vi "CRYO_MASTER_FULL_RUN2.vi"() -> ()   [LabVIEW 2017] (continued)
                n236 = invoke class="TabCtl (strict)" method="Get Image"(error in=errorcluster {"status"=FALSE, "code"=0, "source"=""} ("error in (no error)")) -> (error out=w473:errorcluster, "image data"=w475:T23)  [unwired: 5 in, 4 out]
                n237 = Build Path(base path=w484, name or relative path=w477) -> (appended path=w476:path)
                n238 = call <vilib>:"Write PNG File.vi"("error in (no error)"=w473, "image data"=w475, "path to PNG file"=w476) -> ("error out"=w471:errorcluster)  [unwired: 7 in, 1 out]
              }
            }
            n239 = local write "error out (frontpanel screenshots)"(w464) -> ()
          }
          frame #5 {
            n240 = flat-sequence {
              tunnel: w488 -> [w491]
              tunnel: [w491] -> w487
              tunnel: w489 -> [w506]
              tunnel: w487 -> [w494]
              tunnel: [w493] -> w486
              tunnel: w485 -> [w492]
              frame #0 {
                n241 = property class="TabCtl (strict)"("Val(Sgnl)"=T1."DMMs" ("Value (Signaling)")) -> ()  [unwired: 2 in, 2 out]
              }
              frame #1 {
                w504 = "_" ("string")
                n242 = local read "Cycle #"() -> (w502:u32)
                n243 = call "LV_UNIXTIME.vi"("current time"=w494) -> ("date/time string"=w505:string)  [unwired: 9 in, 1 out]
                n244 = Format Value(format string="%06d", value (0)=w502) -> (output string=w501:string)  [unwired: 1 in]
                n245 = Concatenate Strings(w492, w505, w504, w501, w504, "page6.png" ("string")) -> (w499:string)
                n246 = invoke class="TabCtl (strict)" method="Get Image"(error in=errorcluster {"status"=FALSE, "code"=0, "source"=""} ("error in (no error)")) -> (error out=w495:errorcluster, "image data"=w497:T23)  [unwired: 5 in, 4 out]
                n247 = Build Path(base path=w506, name or relative path=w499) -> (appended path=w498:path)
                n248 = call <vilib>:"Write PNG File.vi"("error in (no error)"=w495, "image data"=w497, "path to PNG file"=w498) -> ("error out"=w493:errorcluster)  [unwired: 7 in, 1 out]
              }
            }
            n249 = local write "error out (frontpanel screenshots)"(w486) -> ()
          }
          frame #6 {
            n250 = flat-sequence {
              tunnel: w510 -> [w513]
              tunnel: [w513] -> w509
              tunnel: w511 -> [w528]
              tunnel: w509 -> [w516]
              tunnel: [w515] -> w508
              tunnel: w507 -> [w514]
              frame #0 {
                n251 = property class="TabCtl (strict)"("Val(Sgnl)"=T1."DIAGRAM" ("Value (Signaling)")) -> ()  [unwired: 2 in, 2 out]
              }
              frame #1 {
                w526 = "_" ("string")
                n252 = local read "Cycle #"() -> (w524:u32)
                n253 = Format Value(format string="%06d", value (0)=w524) -> (output string=w523:string)  [unwired: 1 in]
                n254 = call "LV_UNIXTIME.vi"("current time"=w516) -> ("date/time string"=w527:string)  [unwired: 9 in, 1 out]
                n255 = Concatenate Strings(w514, w527, w526, w523, w526, "page7.png" ("string")) -> (w521:string)
                n256 = invoke class="TabCtl (strict)" method="Get Image"(error in=errorcluster {"status"=FALSE, "code"=0, "source"=""} ("error in (no error)")) -> (error out=w517:errorcluster, "image data"=w519:T23)  [unwired: 5 in, 4 out]
                n257 = Build Path(base path=w528, name or relative path=w521) -> (appended path=w520:path)
                n258 = call <vilib>:"Write PNG File.vi"("error in (no error)"=w517, "image data"=w519, "path to PNG file"=w520) -> ("error out"=w515:errorcluster)  [unwired: 7 in, 1 out]
              }
            }
            n259 = local write "error out (frontpanel screenshots)"(w508) -> ()
          }
          frame #7 {
            n260 = flat-sequence {
              tunnel: w532 -> [w535]
              tunnel: [w535] -> w531
              tunnel: w533 -> [w550]
              tunnel: w531 -> [w538]
              tunnel: [w537] -> w530
              tunnel: w529 -> [w536]
              frame #0 {
                n261 = property class="TabCtl (strict)"("Val(Sgnl)"=T1."CHF" ("Value (Signaling)")) -> ()  [unwired: 2 in, 2 out]
              }
              frame #1 {
                w548 = "_" ("string")
                n262 = local read "Cycle #"() -> (w546:u32)
                n263 = Format Value(format string="%06d", value (0)=w546) -> (output string=w545:string)  [unwired: 1 in]
                n264 = call "LV_UNIXTIME.vi"("current time"=w538) -> ("date/time string"=w549:string)  [unwired: 9 in, 1 out]
                n265 = Concatenate Strings(w536, w549, w548, w545, w548, "page8.png" ("string")) -> (w543:string)
                n266 = invoke class="TabCtl (strict)" method="Get Image"(error in=errorcluster {"status"=FALSE, "code"=0, "source"=""} ("error in (no error)")) -> (error out=w539:errorcluster, "image data"=w541:T23)  [unwired: 5 in, 4 out]
                n267 = Build Path(base path=w550, name or relative path=w543) -> (appended path=w542:path)
                n268 = call <vilib>:"Write PNG File.vi"("error in (no error)"=w539, "image data"=w541, "path to PNG file"=w542) -> ("error out"=w537:errorcluster)  [unwired: 7 in, 1 out]
              }
            }
            n269 = local write "error out (frontpanel screenshots)"(w530) -> ()
          }
          frame #8 {
            n270 = flat-sequence {
              tunnel: w554 -> [w557]
              tunnel: [w557] -> w553
              tunnel: w555 -> [w572]
              tunnel: w553 -> [w560]
              tunnel: [w559] -> w552
              tunnel: w551 -> [w558]
              frame #0 {
                n271 = property class="TabCtl (strict)"("Val(Sgnl)"=T1."(Plc. hld.)" ("Value (Signaling)")) -> ()  [unwired: 2 in, 2 out]
              }
              frame #1 {
                w570 = "_" ("string")
                n272 = local read "Cycle #"() -> (w568:u32)
                n273 = Format Value(format string="%06d", value (0)=w568) -> (output string=w567:string)  [unwired: 1 in]
                n274 = call "LV_UNIXTIME.vi"("current time"=w560) -> ("date/time string"=w571:string)  [unwired: 9 in, 1 out]
                n275 = Concatenate Strings(w558, w571, w570, w567, w570, "page8.png" ("string")) -> (w565:string)
                n276 = invoke class="TabCtl (strict)" method="Get Image"(error in=errorcluster {"status"=FALSE, "code"=0, "source"=""} ("error in (no error)")) -> (error out=w561:errorcluster, "image data"=w563:T23)  [unwired: 5 in, 4 out]
                n277 = Build Path(base path=w572, name or relative path=w565) -> (appended path=w564:path)
                n278 = call <vilib>:"Write PNG File.vi"("error in (no error)"=w561, "image data"=w563, "path to PNG file"=w564) -> ("error out"=w559:errorcluster)  [unwired: 7 in, 1 out]
              }
            }
            n279 = local write "error out (frontpanel screenshots)"(w552) -> ()
          }
          frame #9 {
            n280 = local write "Frontpanel screenshots"(FALSE ("Frontpanel screenshots")) -> ()
          }
        }
        "error out (frontpanel screenshots)" <- w371
        n281 = property class="TabCtl (strict)"("Val(Sgnl)"=w369) -> ()  [unwired: 2 in, 2 out]
      }
      event "Stop Button": Value Change {
        n282 = event-data() -> ()  [unwired: 1 in, 3 out]
      }
    }
    n283 = Wait (ms)(milliseconds to wait=u32 123) -> ()  [unwired: 1 out]
  }
  n284 = while {
    stop <- w579 stop-if-true
    n285 = event shown="[6] \"Take Screenshot! 1\": Value Change" {
      selector: _ -> [_ _ _ _ _ _ _ _ _ _ _]
      dyn-events: _ -> [_ _ _ _ _ _ _ _ _ _ _]
      timeout: _ -> [_ _ _ _ _ _ _ _ _ _ _]
      tunnel: [_ _ _ _ _ _ _ _ _ _ TRUE] -> w579
      tunnel: [errorcluster {"status"=FALSE, "code"=0, "source"=""} ("error out") w583 _ _ _ _ w713 w730 w747 w764 errorcluster {"status"=FALSE, "code"=0, "source"=""} ("error out")] -> w575
      event Timeout {
        n286 = event-data() -> ()  [unwired: 1 in, 3 out]
      }
      event "log/linear 1": Value Change {
        n287 = event-data() -> ()  [unwired: 1 in, 6 out]
        n288 = flat-sequence {
          tunnel: [w584] -> w583
          frame #0 {
            n289 = Boolean To (0,1)(Boolean="log/linear 1") -> (0, 1=w589:i16)
            n290 = control-ref of="Graph 1"() -> (w585:refnum<vi>)
            n291 = property class="XYGraph (strict)"(reference=w585, error in=errorcluster {"status"=FALSE, "code"=0, "source"=""} ("error in (no error)"), "YScale.Mapping Mode"=w589) -> (error out=w587:errorcluster)  [unwired: 1 out]
            n292 = control-ref of="error out (USB6210)"() -> (w588:refnum<vi>)
            n293 = property class="Clust (strict)"(reference=w588, "Val(Sgnl)"=w587) -> (error out=w584:errorcluster)  [unwired: 1 in, 1 out]
          }
        }
      }
      event "log/linear 2": Value Change {
        n294 = event-data() -> ()  [unwired: 1 in, 6 out]
        n295 = flat-sequence {
          frame #0 {
            n296 = Boolean To (0,1)(Boolean="log/linear 2") -> (0, 1=w595:i16)
            n297 = control-ref of="Graph 2"() -> (w593:refnum<vi>)
            n298 = property class="XYGraph (strict)"(reference=w593, error in=errorcluster {"status"=FALSE, "code"=0, "source"=""} ("error in (no error)"), "YScale.Mapping Mode"=w595) -> (error out=w594:errorcluster)  [unwired: 1 out]
            n299 = control-ref of="error out (USB6210)"() -> (w592:refnum<vi>)
            n300 = property class="Clust (strict)"(reference=w592, "Value"=w594) -> ()  [unwired: 1 in, 2 out]
          }
        }
      }
      event "log/linear 3": Value Change {
        n301 = event-data() -> ()  [unwired: 1 in, 6 out]
        n302 = flat-sequence {
          frame #0 {
            n303 = Boolean To (0,1)(Boolean="log/linear 3") -> (0, 1=w601:i16)
            n304 = control-ref of="Graph 3"() -> (w597:refnum<vi>)
            n305 = property class="XYGraph (strict)"(reference=w597, error in=errorcluster {"status"=FALSE, "code"=0, "source"=""} ("error in (no error)"), "YScale.Mapping Mode"=w601) -> (error out=w600:errorcluster)  [unwired: 1 out]
            n306 = control-ref of="error out (USB6210)"() -> (w599:refnum<vi>)
            n307 = property class="Clust (strict)"(reference=w599, "Value"=w600) -> ()  [unwired: 1 in, 2 out]
          }
        }
      }
      event "log/linear 4": Value Change {
        n308 = event-data() -> ()  [unwired: 1 in, 6 out]
        n309 = flat-sequence {
          frame #0 {
            n310 = Boolean To (0,1)(Boolean="log/linear 4") -> (0, 1=w607:i16)
            n311 = control-ref of="Graph 4"() -> (w603:refnum<vi>)
            n312 = property class="XYGraph (strict)"(reference=w603, error in=errorcluster {"status"=FALSE, "code"=0, "source"=""} ("error in (no error)"), "YScale.Mapping Mode"=w607) -> (error out=w606:errorcluster)  [unwired: 1 out]
            n313 = control-ref of="error out (USB6210)"() -> (w605:refnum<vi>)
            n314 = property class="Clust (strict)"(reference=w605, "Value"=w606) -> ()  [unwired: 1 in, 2 out]
          }
        }
      }
      event "Plot selecter LSI218(1)\n    1      2     3     4", "Plot selecter LSI218(2)\n    1      2     3     4", "Plot selecter (USB6210)\n    1      2     3     4", "Plot selecter LSI336 \n     1      2     3     4", "Plot selecter (USB6218)\n    1      2     3     4": Value Change {
        n315 = event-data() -> ()  [unwired: 1 in, 6 out]
        n316 = local read "All Labels (USB6210)"() -> (w625:string[])
        n317 = local read "All Labels (USB6218)"() -> (w614:string[])
        n318 = local read "Labels LSI218 (1)"() -> (w627:string[])
        n319 = local read "Labels LSI218 (2)"() -> (w628:string[])
        n320 = local read "Labels LSI336"() -> (w620:string[])
        n321 = call "BuildPlotLegends_LSI218.vi"("Plot selecter (2)\n    1      2     3     5"="Plot selecter LSI218(2)\n    1      2     3     4", "Plot selecter (1)\n    1      2     3     4"="Plot selecter LSI218(1)\n    1      2     3     4", "Labels (2)"=w628, "Labels (1)"=w627) -> ("Series 4"=w638:string[], "Series 3"=w636:string[], "Series 2"=w634:string[], "Series 1"=w632:string[])  [unwired: 4 in]
        n322 = call "BuildPlotLegends.vi"("Plot selecter \n    1      2     3     4"="Plot selecter (USB6210)\n    1      2     3     4", "AllLabels"=w625) -> ("Series 4"=w637:string[], "Series 3"=w635:string[], "Series 2"=w633:string[], "Series 1"=w631:string[])  [unwired: 6 in]
        n323 = call "BuildPlotLegends.vi"("Plot selecter \n    1      2     3     4"="Plot selecter LSI336 \n     1      2     3     4", "AllLabels"=w620) -> ("Series 4"=w615:string[], "Series 3"=w616:string[], "Series 2"=w617:string[], "Series 1"=w618:string[])  [unwired: 6 in]
        n324 = call "BuildPlotLegends.vi"("Plot selecter \n    1      2     3     4"="Plot selecter (USB6218)\n    1      2     3     4", "AllLabels"=w614) -> ("Series 4"=w610:string[], "Series 3"=w609:string[], "Series 2"=w611:string[], "Series 1"=w612:string[])  [unwired: 6 in]
        n325 = Build Array (concatenate)(w633, w634, w617, w611) -> (w622:string[])
        "Series 2" <- w622
        n326 = Build Array (concatenate)(w635, w636, w616, w609) -> (w623:string[])
        "Series 3" <- w623
        n327 = Build Array (concatenate)(w637, w638, w615, w610) -> (w624:string[])
        "Series 4" <- w624
        n328 = Build Array (concatenate)(w631, w632, w618, w612) -> (w621:string[])
        "Series 1" <- w621
        n329 = stacked-sequence {
          tunnel: [w648 _ _ _] -> w642
          tunnel: [_ w666 _ _] -> w643
          tunnel: [_ _ w683 _] -> w641
          tunnel: [_ _ _ w700] -> w640
          tunnel: w621 -> [w646 _ _ _]
          tunnel: w622 -> [_ w664 _ _]
          tunnel: w623 -> [_ _ w681 _]
          tunnel: w624 -> [_ _ _ w698]
          frame #0 {
            n330 = Array Size(array=w646) -> (size(s)=w650:i32)
            n331 = control-ref of="Graph 1"() -> (w644:refnum<vi>)
            n332 = property class="XYGraph (strict)"(reference=w644) -> ("LegNumRows"=w645:u32)  [unwired: 1 in, 2 out]
            n333 = for {
              N: w645 -> [_]
              tunnel: w644 -> [w659]
              shift-right: [w657] -> w649
              shift-left: errorcluster {"status"=FALSE, "code"=0, "source"=""} ("error in (no error)") -> [w658]
              i -> [w661]
              n334 = property class="XYGraph (strict)"(reference=w659, error in=w658, "Active Plot"=w661, "Plot.Plot Name"="") -> (error out=w657:errorcluster)  [unwired: 1 out]
            }
            n335 = for {
              N: w650 -> [_]
              tunnel: w644 -> [w655]
              shift-right: [w653] -> w648
              shift-left: w649 -> [w654]
              tunnel: w646 -> [w652] mode=indexing
              i -> [w656]
              n336 = property class="XYGraph (strict)"(reference=w655, error in=w654, "Active Plot"=w656, "Plot.Plot Name"=w652, "Plot.Visible?"=TRUE ("Plot.Visible")) -> (error out=w653:errorcluster)  [unwired: 1 out]
            }
          }
          frame #1 {
            n337 = Array Size(array=w664) -> (size(s)=w668:i32)
            n338 = control-ref of="Graph 2"() -> (w663:refnum<vi>)
            n339 = property class="XYGraph (strict)"(reference=w663) -> ("LegNumRows"=w662:u32)  [unwired: 1 in, 2 out]
            n340 = for {
              N: w662 -> [_]
              shift-right: [w675] -> w667
              shift-left: errorcluster {"status"=FALSE, "code"=0, "source"=""} ("error in (no error)") -> [w676]
              tunnel: w663 -> [w674]
              i -> [w678]
              n341 = property class="XYGraph (strict)"(reference=w674, error in=w676, "Active Plot"=w678, "Plot.Plot Name"="") -> (error out=w675:errorcluster)  [unwired: 1 out]
            }
            n342 = for {
              N: w668 -> [_]
              shift-right: [w671] -> w666
              shift-left: w667 -> [w672]
              tunnel: w664 -> [w670] mode=indexing
              tunnel: w663 -> [w669]
              i -> [w673]
              n343 = property class="XYGraph (strict)"(reference=w669, error in=w672, "Active Plot"=w673, "Plot.Plot Name"=w670) -> (error out=w671:errorcluster)  [unwired: 1 out]
            }
          }
          frame #2 {
            n344 = Array Size(array=w681) -> (size(s)=w685:i32)
            n345 = control-ref of="Graph 3"() -> (w679:refnum<vi>)
            n346 = property class="XYGraph (strict)"(reference=w679) -> ("LegNumRows"=w680:u32)  [unwired: 1 in, 2 out]
            n347 = for {
              N: w680 -> [_]
              tunnel: w679 -> [w693]
              shift-right: [w691] -> w684
              shift-left: errorcluster {"status"=FALSE, "code"=0, "source"=""} ("error in (no error)") -> [w692]
              i -> [w695]
              n348 = property class="XYGraph (strict)"(reference=w693, error in=w692, "Active Plot"=w695, "Plot.Plot Name"="") -> (error out=w691:errorcluster)  [unwired: 1 out]
            }
            n349 = for {
              N: w685 -> [_]
              tunnel: w679 -> [w689]
              shift-right: [w687] -> w683
              shift-left: w684 -> [w688]
              tunnel: w681 -> [w686] mode=indexing
              i -> [w690]
              n350 = property class="XYGraph (strict)"(reference=w689, error in=w688, "Active Plot"=w690, "Plot.Plot Name"=w686) -> (error out=w687:errorcluster)  [unwired: 1 out]
            }
          }
          frame #3 {
            n351 = Array Size(array=w698) -> (size(s)=w702:i32)
            n352 = control-ref of="Graph 4"() -> (w696:refnum<vi>)
            n353 = property class="XYGraph (strict)"(reference=w696) -> ("LegNumRows"=w697:u32)  [unwired: 1 in, 2 out]
            n354 = for {
              N: w697 -> [_]
              tunnel: w696 -> [w710]
              shift-right: [w708] -> w701
              shift-left: errorcluster {"status"=FALSE, "code"=0, "source"=""} ("error in (no error)") -> [w709]
              i -> [w712]
              n355 = property class="XYGraph (strict)"(reference=w710, error in=w709, "Active Plot"=w712, "Plot.Plot Name"="") -> (error out=w708:errorcluster)  [unwired: 1 out]
            }
            n356 = for {
              N: w702 -> [_]
              tunnel: w696 -> [w706]
              shift-right: [w704] -> w700
              shift-left: w701 -> [w705]
              tunnel: w698 -> [w703] mode=indexing
              i -> [w707]
              n357 = property class="XYGraph (strict)"(reference=w706, error in=w705, "Active Plot"=w707, "Plot.Plot Name"=w703) -> (error out=w704:errorcluster)  [unwired: 1 out]
            }
          }
        }
        n358 = Merge Errors(w642, w643, w641, w640) -> (→"Plot errors":errorcluster)
      }
      event "Take Screenshot! 1": Value Change {
        n359 = event-data() -> ()  [unwired: 1 in, 6 out]
        n360 = flat-sequence {
          tunnel: [w714] -> w713
          frame #0 {
            n361 = flat-sequence {
              tunnel: [w715] -> w714
              frame #0 {
                w724 = "_" ("string")
                n362 = Get Date/Time In Seconds() -> (seconds since 1Jan1904=w721:timestamp)
                n363 = local read "RUN Identifier"() -> (w726:string)
                n364 = call "LV_UNIXTIME.vi"("current time"=w721) -> ("date/time string"=w725:string)  [unwired: 9 in, 1 out]
                n365 = control-ref of="Graph 1"() -> (w720:refnum<vi>)
                n366 = Concatenate Strings(w726, w724, w725, w724, "FIle suffix 1", ".png" ("string")) -> (w728:string)
                n367 = local read "Base Path"() -> (w727:path)
                n368 = invoke class="XYGraph (strict)" method="Get Image"(reference=w720, error in=errorcluster {"status"=FALSE, "code"=0, "source"=""} ("error in (no error)")) -> (error out=w716:errorcluster, "image data"=w719:T23)  [unwired: 4 in, 4 out]
                n369 = Build Path(base path=w727, name or relative path=w728) -> (appended path=w718:path)
                n370 = call <vilib>:"Write PNG File.vi"("error in (no error)"=w716, "image data"=w719, "path to PNG file"=w718) -> ("error out"=w715:errorcluster)  [unwired: 7 in, 1 out]
              }
              frame #1 {
                n371 = local write "Take Screenshot! 1"(FALSE ("Take Screenshot! 1")) -> ()
              }
            }
          }
        }
      }
      event "Take Screenshot! 2": Value Change {
        n372 = event-data() -> ()  [unwired: 1 in, 6 out]
        n373 = flat-sequence {
          tunnel: [w731] -> w730
          frame #0 {
            n374 = flat-sequence {
              tunnel: [w737] -> w731
              frame #0 {
                w741 = "_" ("string")
                n375 = Get Date/Time In Seconds() -> (seconds since 1Jan1904=w738:timestamp)
                n376 = local read "RUN Identifier"() -> (w743:string)
                n377 = call "LV_UNIXTIME.vi"("current time"=w738) -> ("date/time string"=w742:string)  [unwired: 9 in, 1 out]
                n378 = control-ref of="Graph 2"() -> (w732:refnum<vi>)
                n379 = Concatenate Strings(w743, w741, w742, w741, "FIle suffix 2", ".png" ("string")) -> (w745:string)
                n380 = local read "Base Path"() -> (w744:path)
                n381 = invoke class="XYGraph (strict)" method="Get Image"(reference=w732, error in=errorcluster {"status"=FALSE, "code"=0, "source"=""} ("error in (no error)")) -> (error out=w736:errorcluster, "image data"=w734:T23)  [unwired: 4 in, 4 out]
                n382 = Build Path(base path=w744, name or relative path=w745) -> (appended path=w733:path)
                n383 = call <vilib>:"Write PNG File.vi"("error in (no error)"=w736, "image data"=w734, "path to PNG file"=w733) -> ("error out"=w737:errorcluster)  [unwired: 7 in, 1 out]
              }
              frame #1 {
                n384 = local write "Take Screenshot! 2"(FALSE ("Take Screenshot! 1")) -> ()
              }
            }
          }
        }
      }
      event "Take Screenshot! 3": Value Change {
        n385 = event-data() -> ()  [unwired: 1 in, 6 out]
        n386 = flat-sequence {
          tunnel: [w748] -> w747
          frame #0 {
            n387 = flat-sequence {
              tunnel: [w750] -> w748
              frame #0 {
                w758 = "_" ("string")
                n388 = Get Date/Time In Seconds() -> (seconds since 1Jan1904=w756:timestamp)
                n389 = local read "RUN Identifier"() -> (w760:string)
                n390 = call "LV_UNIXTIME.vi"("current time"=w756) -> ("date/time string"=w759:string)  [unwired: 9 in, 1 out]
                n391 = control-ref of="Graph 3"() -> (w753:refnum<vi>)
                n392 = Concatenate Strings(w760, w758, w759, w758, "FIle suffix 3", ".png" ("string")) -> (w762:string)
                n393 = local read "Base Path"() -> (w761:path)
                n394 = invoke class="XYGraph (strict)" method="Get Image"(reference=w753, error in=errorcluster {"status"=FALSE, "code"=0, "source"=""} ("error in (no error)")) -> (error out=w751:errorcluster, "image data"=w749:T23)  [unwired: 4 in, 4 out]
                n395 = Build Path(base path=w761, name or relative path=w762) -> (appended path=w754:path)
                n396 = call <vilib>:"Write PNG File.vi"("error in (no error)"=w751, "image data"=w749, "path to PNG file"=w754) -> ("error out"=w750:errorcluster)  [unwired: 7 in, 1 out]
              }
              frame #1 {
                n397 = local write "Take Screenshot! 3"(FALSE ("Take Screenshot! 1")) -> ()
              }
            }
          }
        }
      }
      event "Take Screenshot! 4": Value Change {
        n398 = event-data() -> ()  [unwired: 1 in, 6 out]
        n399 = flat-sequence {
          tunnel: [w765] -> w764
          frame #0 {
            n400 = flat-sequence {
              tunnel: [w768] -> w765
              frame #0 {
                w775 = "_" ("string")
                n401 = Get Date/Time In Seconds() -> (seconds since 1Jan1904=w773:timestamp)
                n402 = local read "RUN Identifier"() -> (w777:string)
                n403 = call "LV_UNIXTIME.vi"("current time"=w773) -> ("date/time string"=w776:string)  [unwired: 9 in, 1 out]
                n404 = control-ref of="Graph 4"() -> (w769:refnum<vi>)
                n405 = Concatenate Strings(w777, w775, w776, w775, "FIle suffix 4", ".png" ("string")) -> (w779:string)
                n406 = local read "Base Path"() -> (w778:path)
                n407 = invoke class="XYGraph (strict)" method="Get Image"(reference=w769, error in=errorcluster {"status"=FALSE, "code"=0, "source"=""} ("error in (no error)")) -> (error out=w766:errorcluster, "image data"=w770:T23)  [unwired: 4 in, 4 out]
                n408 = Build Path(base path=w778, name or relative path=w779) -> (appended path=w771:path)
                n409 = call <vilib>:"Write PNG File.vi"("error in (no error)"=w766, "image data"=w770, "path to PNG file"=w771) -> ("error out"=w768:errorcluster)  [unwired: 7 in, 1 out]
              }
              frame #1 {
                n410 = local write "Take Screenshot! 4"(FALSE ("Take Screenshot! 1")) -> ()
              }
            }
          }
        }
      }
      event "Stop Button": Value Change {
        n411 = event-data() -> ()  [unwired: 1 in, 6 out]
      }
    }
    "error out (graph operations)" <- w575
    n412 = local write "Take Screenshot! 1"(FALSE ("Take Screenshot! 1")) -> ()
    n413 = local write "Take Screenshot! 2"(FALSE ("Take Screenshot! 1")) -> ()
    n414 = Wait (ms)(milliseconds to wait=u32 1000) -> ()  [unwired: 1 out]
    n415 = local write "Take Screenshot! 3"(FALSE ("Take Screenshot! 1")) -> ()
    n416 = local write "Take Screenshot! 4"(FALSE ("Take Screenshot! 1")) -> ()
  }
  n417 = while {
    i -> [w787]
    stop <- w784 stop-if-true
    n418 = Equal?(x=w787, y=0) -> (x = y?=w785:bool)
    n419 = case shown="True" w785 {
      frame False {
      }
      frame True {
        n420 = property on="Agilent\nIntialized?" class="Bool (strict)"("Val(Sgnl)"=FALSE ("Value (Signaling)")) -> ()  [unwired: 2 in, 2 out]
      }
    }
    n421 = Wait (ms)(milliseconds to wait=u32 123) -> ()  [unwired: 1 out]
    n422 = event shown="[4] \"V_lim_up (V)\", \"V_lim_low (V)\": Value Change" {
      selector: _ -> [_ _ _ _ _]
      dyn-events: _ -> [_ _ _ _ _]
      timeout: _ -> [_ _ _ _ _]
      tunnel: [FALSE ("Value (Signaling)") TRUE ("Value (Signaling)") _ _ _] -> w784
      tunnel: "VISA (Agilent 34402)" -> [_ _ w793 w796 _]
      event Timeout {
        n423 = event-data() -> ()  [unwired: 1 in, 3 out]
      }
      event "Stop Button": Value Change {
        n424 = event-data() -> ()  [unwired: 1 in, 3 out]
      }
      event "Initialize (Agilent)": Value Change {
        n425 = event-data() -> ()  [unwired: 1 in, 3 out]
        n426 = property on="Agilent\nIntialized?" class="Bool (strict)"("Val(Sgnl)"=TRUE ("Value (Signaling)")) -> ()  [unwired: 2 in, 2 out]
        n427 = call "Initialize.vi"("error in (no error)"=errorcluster {"status"=FALSE, "code"=0, "source"=""}, "VISA resource name"=w793) -> ("error out"=→"error out (Agilent)":errorcluster)  [unwired: 8 in, 1 out]
      }
      event "OUTPUT \nKenwood", "Kenwood set V (V)": Value Change {
        n428 = local read "Agilent\nIntialized?"() -> (w795:bool)
        n429 = event-data() -> ()  [unwired: 1 in, 3 out]
        n430 = case shown="True" w795 {
          tunnel: w796 -> [_ w802]
          frame False {
          }
          frame True {
            w804 = u16 0 items=["DC", "Sine", "Square", "Triangle", "Ramp", "Pulse", "Noise", "Sinc", "Negative Ramp", "Exponential Rise", "Exponential Fall", "Cardiac"] ("Waveform Function (1: Sine)")
            n431 = xnode "Formula"("X1"="Kenwood set V (V)") -> ("Result"=w797:dbl)  [unwired: 1 in, 1 out]
            n432 = call "Configure Standard Waveform.vi"("DC Offset (0.00 V)"=w797, "Frequency (1000 Hz)"=1.0, "error in (no error)"=errorcluster {"status"=FALSE, "code"=0, "source"=""}, "Amplitude (1)"=1.0, "Waveform Function (1: Sine)"=w804, "VISA resource name"=w802) -> ("error out"=w806:errorcluster, "VISA resource name out"=w807:refnum<visa-resource-name>)  [unwired: 4 in]
            n433 = call "Enable Output.vi"("error in (no error)"=w806, "Enable Output  (T: Enable)"="OUTPUT \nKenwood", "VISA resource name"=w807) -> ("error out"=w800:errorcluster)  [unwired: 7 in, 1 out]
            n434 = local write "error out (Agilent)"(w800) -> ()
          }
        }
      }
      event "V_lim_up (V)", "V_lim_low (V)": Value Change {
        n435 = event-data() -> ()  [unwired: 1 in, 3 out]
        n436 = property on="Kenwood set V (V)" class="DigNum (strict)"("Minimum"="V_lim_low (V)", "Maximum"="V_lim_up (V)") -> ()  [unwired: 2 in, 2 out]
      }
    }
  }
  n437 = while {
    stop <- w819 stop-if-true
    n438 = Wait (ms)(milliseconds to wait=u32 101) -> ()  [unwired: 1 out]
    n439 = event shown="[2] Timeout" {
      selector: _ -> [_ _ _]
      dyn-events: _ -> [_ _ _]
      timeout: _ -> [_ _ _]
      tunnel: [FALSE TRUE FALSE] -> w819
      event "Initialize (DMMs)": Value Change {
        w822 = T4 [] ("Value (Signaling)")
        n440 = event-data() -> ()  [unwired: 1 in, 3 out]
        n441 = property on="Graph DMMs 1" class="XYGraph (strict)"("Val(Sgnl)"=w822) -> ()  [unwired: 2 in, 2 out]
        n442 = property on="Graph DMMs 2" class="XYGraph (strict)"("Val(Sgnl)"=w822) -> ()  [unwired: 2 in, 2 out]
      }
      event "Stop Button": Value Change {
        n443 = event-data() -> ()  [unwired: 1 in, 3 out]
      }
      event Timeout {
        n444 = event-data() -> ()  [unwired: 1 in, 3 out]
      }
    }
  }
  n445 = Obtain Notifier(name (unnamed)="stop notifier", notification data type=w15, create if not found? (T)=w15, error in (no error)=errorcluster {"status"=FALSE, "code"=0, "source"=""}) -> (notifier out=w3:refnum<notifier>, error out=w2:errorcluster)  [unwired: 1 out]
  n446 = while {
    shift-right: [w922] -> w38
    shift-left: refnum<class "USBData.lvclass"> refnum ("USBData.lvclass") -> [w925]
    shift-right: [w918] -> w37
    shift-left: w4 -> [w924]
    tunnel: "Base Path" -> [w862]
    shift-right: [w900] -> w32
    shift-left: errorcluster {"status"=FALSE, "code"=0, "source"=""} ("error in (no error)") -> [w916]
    shift-right: [w901] -> w33
    shift-left: refnum<class "LSI218Data.lvclass"> refnum ("LSI218Data.lvclass") -> [w915]
    shift-right: [w888] -> w29
    shift-left: refnum<class "LSI336Data.lvclass"> refnum ("LSI336Data.lvclass") -> [w897]
    shift-right: [w887] -> w28
    shift-left: w19 -> [w896]
    shift-right: [w876] -> _
    shift-left: w4 -> [w877]
    shift-right: [w866] -> w23
    shift-left: refnum<class "USBData.lvclass"> refnum ("USBData.lvclass") -> [w874]
    shift-right: [w865] -> w22
    shift-left: errorcluster {"status"=FALSE, "code"=0, "source"=""} ("error in (no error)") -> [w873]
    shift-right: [w861] -> _
    shift-left: w19 -> [w860]
    tunnel: w3 -> [w829]
    tunnel: w2 -> [w828]
    tunnel: [w826] -> w11
    tunnel: [w825] -> w10
    i -> [w837]
    stop <- "Stop Button" stop-if-true
    w883 = u32 24 ("Number of Rows")
    w893 = T25 [] ("appended array")
    w910 = T25 [] ("appended array")
    n447 = local read "LSI218Settings(A-F)"() -> (w852:T3)
    n448 = control-ref of="Plot selecter LSI218(2)\n    1      2     3     4"() -> (w881:refnum<vi>)
    n449 = control-ref of="Plot selecter LSI218(1)\n    1      2     3     4"() -> (w882:refnum<vi>)
    n450 = control-ref of="Plot selecter LSI336 \n     1      2     3     4"() -> (w880:refnum<vi>)
    n451 = property on="Property Node" class="Arr (strict)"(reference=w881, "Number of Rows"=w883) -> ()  [unwired: 1 in, 2 out]
    n452 = property on="Property Node" class="Arr (strict)"(reference=w882, "Number of Rows"=w883) -> ()  [unwired: 1 in, 2 out]
    n453 = local read "LSI336Settings(X,Y)"() -> (w850:T3)
    n454 = Array Size(array=w852) -> (size(s)=w851:i32)
    n455 = property on="Property Node" class="Arr (strict)"(reference=w880, "Number of Rows"=u32 8) -> ()  [unwired: 1 in, 2 out]
    n456 = Multiply(x="Measurement Interval (s)", y=u32 1000) -> (x*y=w919:dbl)
    n457 = Wait (ms)(milliseconds to wait=w919) -> ()  [unwired: 1 out]
    n458 = for {
      N: w851 -> [_]
      tunnel: w852 -> [w936] mode=indexing
      tunnel: [w935] -> w848 mode=concatenating
      n459 = Unbundle By Name(w936) -> ("SensorLocations"=w935:T18)
    }
    n460 = for {
      tunnel: w850 -> [w934] mode=indexing
      tunnel: [w933] -> w849 mode=concatenating
      n461 = Unbundle By Name(w934) -> ("SensorLocations"=w933:T18)
    }
    n462 = Quotient & Remainder(x=w837, y="Screenshots interval") -> (x-y*floor(x/y)=w835:i64)  [unwired: 1 out]
    n463 = Equal?(x=w837, y=0) -> (x = y?=w830:bool)
    n464 = case shown="True" w830 {
      tunnel: w925 -> [w1991 w2014]
      tunnel: w924 -> [w1985 w2012]
      tunnel: w837 -> [w1976 _]
      tunnel: [w1983 w2009] -> w918
      tunnel: [w1980 w2008] -> w875
      tunnel: [w1981 w2007] -> w922
      tunnel: [w1971 w2002] -> w923
      tunnel: w862 -> [_ w2001]
      tunnel: [w1970 w1998] -> w857
      frame False {
        n465 = call-dynamic "USBData_measure.vi"("USBData in"=w1991, "DAQ sample #"=i64 5, "DAQ timeout"=100.0 ("DAQ timeout (def: 100)"), "MeasurementIndex"=w1976, "error in (no error)"=w1985, "save every ... measurements"="Record interval") -> ("USBData out"=w1990:refnum<class "USBData.lvclass">, "TimeMeasuremeent"=w1987:timestamp, "Status"=→"USB6210 Status":T6, "LastDataAcquired"=w1972:dbl[], "error out"=w1986:errorcluster)  [unwired: 3 in, 2 out]
        "Time of Last Measurement (USB6210)" <- w1987
        "Last Vol\n(USB6210)" <- w1972
        n466 = call-dynamic "USBData_convert.vi"("Save every ... measurements"="Record interval", "MeasurementIndex"=w1976, "error in (no error)"=w1986, "LastDataAcquired"=w1972, "TimeMeasuremeent"=w1987, "USBData in"=w1990) -> ("error out"=w1984:errorcluster, "LeakDet_FULL"=w1979:dbl, "LastDataConverted"=w1973:dbl[], "USBData out"=w1982:refnum<class "USBData.lvclass">)  [unwired: 2 in]
        n467 = call "USBData_read.vi"("USBData in"=w1982, "error in (no error)"=w1984) -> ("Status"=w1974:T6, "USBData out"=w1981:refnum<class "USBData.lvclass">, "Data"=w1980:T26, "Basic"=w1971:T27, "error out"=w1983:errorcluster)  [unwired: 2 in, 2 out]
        n468 = local write "USB6210 Status"(w1974) -> ()
        n469 = Unbundle By Name(w1971) -> ("ReadLeakDet?"=w1978:bool)
        n470 = Unbundle By Name(w1971) -> ("Labels"=w1970:string[])
        n471 = case shown="False" w1978 {
          tunnel: w1973 -> [w1992 w1995]
          tunnel: w1979 -> [_ w1994]
          tunnel: [w1992 w1993] -> w1977
          frame False {
          }
          frame True {
            n472 = Build Array (concatenate)(w1995, w1994) -> (w1993:dbl[])
          }
        }
        "Last Data \n(USB6210)" <- w1977
      }
      frame True {
        n473 = local read "RUN Identifier"() -> (w1996:string)
        n474 = call-dynamic "USBData_initialize.vi"("USBData in"=w2014, "SeriesSetting"="USB6210 Config", "BasePath"=w2001, "RunIdentifier"=w1996, "FileName"="InstName (USB6210)", "error in (no error)"=w2012) -> ("Status"=w1997:T6, "USBData out"=w2010:refnum<class "USBData.lvclass">, "error out"=w2011:errorcluster)  [unwired: 5 in, 2 out]
        n475 = local write "USB6210 Status"(w1997) -> ()
        n476 = call "USBData_read.vi"("USBData in"=w2010, "error in (no error)"=w2011) -> ("Status"=w2000:T6, "USBData out"=w2007:refnum<class "USBData.lvclass">, "Data"=w2008:T26, "Basic"=w2002:T27, "error out"=w2009:errorcluster)  [unwired: 2 in, 2 out]
        n477 = local write "USB6210 Status"(w2000) -> ()
        n478 = Unbundle By Name(w2002) -> ("ReadLeakDet?"=w2006:bool, "Labels"=w1998:string[])
        n479 = Array Size(array=w1998) -> (size(s)=w2005:i32)
        n480 = case shown="True" w2006 {
          tunnel: w2005 -> [w2015 w2017]
          tunnel: [w2015 w2016] -> w2003
          frame False {
          }
          frame True {
            n481 = Add(x=w2017, y=1) -> (x+y=w2016:i32)
          }
        }
        n482 = Initialize Array(TRUE ("Activate 2"), w2003) -> ()  [unwired: 1 out]
      }
    }
    "error out (USB6210)" <- w918
    n483 = case shown="False" w830 {
      tunnel: [w1507 w1534] -> w865
      tunnel: [w1504 w1533] -> w872
      tunnel: [w1505 w1532] -> w866
      tunnel: [w1496 w1527] -> w871
      tunnel: [w1495 w1525] -> _
      tunnel: w874 -> [w1494 w1523]
      tunnel: w862 -> [_ w1522]
      tunnel: w873 -> [w1493 w1521]
      tunnel: w837 -> [w1492 _]
      frame False {
        n484 = local read "Record interval"() -> (w1491:i64)
        n485 = call-dynamic "USBData_measure.vi"("USBData in"=w1494, "DAQ sample #"=i64 5, "DAQ timeout"=100.0 ("DAQ timeout (def: 100)"), "MeasurementIndex"=w1492, "error in (no error)"=w1493, "save every ... measurements"=w1491) -> ("USBData out"=w1513:refnum<class "USBData.lvclass">, "TimeMeasuremeent"=w1510:timestamp, "Status"=→"USB6218 Status":T6, "LastDataAcquired"=w1497:dbl[], "error out"=w1509:errorcluster)  [unwired: 3 in, 2 out]
        "Time of Last Measurement (USB6218)" <- w1510
        "Last Vol \n(USB6218)" <- w1497
        n486 = call-dynamic "USBData_convert.vi"("Save every ... measurements"=w1491, "MeasurementIndex"=w1492, "error in (no error)"=w1509, "LastDataAcquired"=w1497, "TimeMeasuremeent"=w1510, "USBData in"=w1513) -> ("error out"=w1508:errorcluster, "LeakDet_FULL"=w1503:dbl, "LastDataConverted"=w1498:dbl[], "USBData out"=w1506:refnum<class "USBData.lvclass">)  [unwired: 2 in]
        n487 = call "USBData_read.vi"("USBData in"=w1506, "error in (no error)"=w1508) -> ("Status"=w1499:T6, "USBData out"=w1505:refnum<class "USBData.lvclass">, "Data"=w1504:T26, "Basic"=w1496:T27, "error out"=w1507:errorcluster)  [unwired: 2 in, 2 out]
        n488 = local write "USB6218 Status"(w1499) -> ()
        n489 = Unbundle By Name(w1496) -> ("ReadLeakDet?"=w1502:bool)
        n490 = Unbundle By Name(w1496) -> ("Labels"=w1495:string[])
        n491 = case shown="True" w1502 {
          tunnel: w1498 -> [w1514 w1517]
          tunnel: w1503 -> [_ w1516]
          tunnel: [w1514 w1515] -> w1501
          frame False {
          }
          frame True {
            n492 = Build Array (concatenate)(w1517, w1516) -> (w1515:dbl[])
          }
        }
        "Last Data \n(USB6218)" <- w1501
      }
      frame True {
        n493 = local read "RUN Identifier"() -> (w1518:string)
        n494 = call-dynamic "USBData_initialize.vi"("USBData in"=w1523, "SeriesSetting"="USB6218 Config", "BasePath"=w1522, "RunIdentifier"=w1518, "FileName"="InstName (USB6218)", "error in (no error)"=w1521) -> ("Status"=w1519:T6, "USBData out"=w1535:refnum<class "USBData.lvclass">, "error out"=w1536:errorcluster)  [unwired: 5 in, 2 out]
        n495 = local write "USB6218 Status"(w1519) -> ()
        n496 = call "USBData_read.vi"("USBData in"=w1535, "error in (no error)"=w1536) -> ("Status"=w1526:T6, "USBData out"=w1532:refnum<class "USBData.lvclass">, "Data"=w1533:T26, "Basic"=w1527:T27, "error out"=w1534:errorcluster)  [unwired: 2 in, 2 out]
        n497 = local write "USB6218 Status"(w1526) -> ()
        n498 = Unbundle By Name(w1527) -> ("ReadLeakDet?"=w1531:bool, "Labels"=w1525:string[])
        n499 = Array Size(array=w1525) -> (size(s)=w1530:i32)
        n500 = case shown="True" w1531 {
          tunnel: w1530 -> [w1537 w1539]
          tunnel: [w1537 w1538] -> w1528
          frame False {
          }
          frame True {
            n501 = Add(x=w1539, y=1) -> (x+y=w1538:i32)
          }
        }
        n502 = Initialize Array(TRUE ("Activate 2"), w1528) -> ()  [unwired: 1 out]
      }
    }
    "error out (USB6218)" <- w865
    n503 = case shown="True" w830 {
      frame False {
      }
      frame True {
        n504 = local read "RUN label"() -> (w927:string)
        n505 = Get Date/Time In Seconds() -> (seconds since 1Jan1904=w931:timestamp)
        n506 = call "LV_UNIXTIME.vi"("current time"=w931) -> ("date/time string"=w930:string)  [unwired: 9 in, 1 out]
        n507 = Concatenate Strings(w930, "_" ("string"), w927) -> (→"RUN Identifier" →"RUN Identifier 2" →"RUN Identifier 3" →"RUN Identifier 4" →"RUN Identifier 5" →"RUN Identifier 6" →"RUN Identifier 7":string)
      }
    }
    n508 = Equal?(x=w835, y=i64 0) -> (x = y?=w832:bool)
    n509 = local read "LastData (LSI218)"() -> (w846:dbl[])
    n510 = local read "Last Data \nLSI336"() -> (w845:dbl[])
    n511 = And(x="Analog Out ON?", y=w830) -> (x .and. y?=w863:bool)
    n512 = case shown="True" w863 {
      tunnel: w862 -> [_ w1310]
      tunnel: [w1286 w1301] -> w861
      tunnel: w860 -> [w1286 w1300]
      frame False {
      }
      frame True {
        w1293 = "_raw" ("string")
        w1317 = 10.0 ("V_lim_max")
        w1316 = 0.0 ("V_lim_min")
        w1315 = -1 items=["Default"=-1, "RSE"=10083, "Differential"=10106, "Pseudodifferential"=12529] ("output terminal configuration")
        w1314 = 10348 items=["Volts"=10348, "From Custom Scale"=10065] ("units")
        n513 = local read "RUN Identifier"() -> (w1299:string)
        n514 = Concatenate Strings(w1299, "_AO" ("string")) -> (w1319:string)
        n515 = Concatenate Strings(w1299, "_", "USB_AOUT.csv" ("string")) -> (w1311:string)
        n516 = Array To Cluster(array="AOUT Labels") -> (cluster=w1297:T28)
        n517 = Unbundle By Name(w1297) -> ("AOUT Labels[0]"=w1296:string, "AOUT Labels[1]"=w1294:string)
        n518 = Build Path(base path=w1310, name or relative path=w1311) -> (appended path=w1307:path)
        n519 = Concatenate Strings(w1296, w1293) -> (w1295:string)
        n520 = Concatenate Strings(w1294, w1293) -> (w1292:string)
        n521 = Open/Create/Replace File(file path (use dialog)=w1307, operation (0:open)=T24."open or create") -> (refnum out=w1305:refnum<file>)  [unwired: 4 in, 2 out]
        n522 = Build Array(w1296, w1294, w1295, w1292) -> (w1303:string[])
        n523 = call "FileIntialize.vi"("Error In"=w1300, "Labels"=w1303, "refnum in"=w1305) -> ("Error Out"=w1302:errorcluster, "File Refnum"=→"File Refn USB AO":refnum<file>)  [unwired: 7 in]
        n524 = call <vilib>:"DAQmx Create Task.vi"("new task name"=w1319, "auto cleanup"=FALSE, "error in"=w1302) -> ("task out"=w1318:refnum<k21>, "error out"=w1320:errorcluster)  [unwired: 11 in]
        n525 = Index Array(array="AOUT assignment", index #1=0 ("index"), index #2=1 ("index")) -> (element #1=w1289:tag, element #2=w1287:tag)
        n526 = call-poly <vilib>:"DAQmx Create Virtual Channel.vi"("task in"=w1318, "maximum value"=w1317, "minimum value"=w1316, "output terminal configuration"=w1315, "physical channels"=w1289, "units"=w1314, "error in"=w1320) -> ("task out"=w1322:refnum<k21>, "error out"=w1323:errorcluster)  [unwired: 7 in]
        n527 = call-poly <vilib>:"DAQmx Create Virtual Channel.vi"("task in"=w1322, "maximum value"=w1317, "minimum value"=w1316, "physical channels"=w1287, "error in"=w1323) -> ("task out"=w1325:refnum<k21>, "error out"=w1324:errorcluster)  [unwired: 9 in]
        n528 = call <vilib>:"DAQmx Start Task.vi"("task/channels in"=w1325, "error in"=w1324) -> ("task out"=→"AO task out":refnum<k21>, "error out"=w1301:errorcluster)  [unwired: 12 in]
      }
    }
    "error out (USB6210/6218 AOUT)" <- w861
    n529 = And(x=w832, y="Automatic \nScreenshots?") -> (x .and. y?=w831:bool)
    n530 = Build Array (concatenate)(w846, w845) -> (w844:dbl[])
    "AllTemperatures" <- w844
    n531 = Build Array (concatenate)(w848, w849) -> (w847:T18)
    "TempSensorsLocations" <- w847
    n532 = case shown="True" w831 {
      frame False {
      }
      frame True {
        n533 = flat-sequence {
          frame #0 {
            n534 = property on="Frontpanel screenshots" class="Bool (strict)"("Val(Sgnl)"=TRUE ("Value (Signaling)")) -> ()  [unwired: 2 in, 2 out]
          }
        }
      }
    }
    n535 = flat-sequence {
      tunnel: w844 -> [w937]
      tunnel: w847 -> [w938]
      tunnel: w839 -> [w1190]
      tunnel: w838 -> [w1189]
      frame #0 {
        n536 = stacked-sequence {
          tunnel: w938 -> [w943 w948 w953 w958 w963 w968 w973 w978 w983 w988 w993 w998 w1003 w1008 w1013 w1018 w1023 w1028 w1033 w1038 w1043 w1048 w1053 w1058 w1063 w1068 w1073 w1078 w1083 w1088 w1093 w1098 w1103 w1108 w1113 w1118 w1123 w1128 w1133 w1138 w1143 w1148 w1153 w1158 w1163 w1168 w1173 w1178 w1183 w1188]
          tunnel: w937 -> [w941 w946 w951 w956 w961 w966 w971 w976 w981 w986 w991 w996 w1001 w1006 w1011 w1016 w1021 w1026 w1031 w1036 w1041 w1046 w1051 w1056 w1061 w1066 w1071 w1076 w1081 w1086 w1091 w1096 w1101 w1106 w1111 w1116 w1121 w1126 w1131 w1136 w1141 w1146 w1151 w1156 w1161 w1166 w1171 w1176 w1181 w1186]
          frame #0 {
            n537 = Search 1D Array(1D array=w943, element=T14."T3He1-1" ("SensorLocations")) -> (index of element=w940:i32)  [unwired: 1 in]
            n538 = Index Array(array=w941, index=w940) -> (element=→"T3He1-1":dbl)
          }
          frame #1 {
            n539 = Search 1D Array(1D array=w948, element=T14."T3He1-2" ("SensorLocations")) -> (index of element=w945:i32)  [unwired: 1 in]
            n540 = Index Array(array=w946, index=w945) -> (element=→"T3He1-2":dbl)
          }
          frame #2 {
            n541 = Search 1D Array(1D array=w953, element=T14."T3He1-3" ("SensorLocations")) -> (index of element=w950:i32)  [unwired: 1 in]
            n542 = Index Array(array=w951, index=w950) -> (element=→"T3He1-3":dbl)
          }
          frame #3 {
            n543 = Search 1D Array(1D array=w958, element=T14."T3He1-4" ("SensorLocations")) -> (index of element=w955:i32)  [unwired: 1 in]
            n544 = Index Array(array=w956, index=w955) -> (element=→"T3He1-4":dbl)
          }
          frame #4 {
            n545 = Search 1D Array(1D array=w963, element=T14."T3He2-1" ("SensorLocations")) -> (index of element=w960:i32)  [unwired: 1 in]
            n546 = Index Array(array=w961, index=w960) -> (element=→"T3He2-1":dbl)
          }
          frame #5 {
            n547 = Search 1D Array(1D array=w968, element=T14."T3He2-2" ("SensorLocations")) -> (index of element=w965:i32)  [unwired: 1 in]
            n548 = Index Array(array=w966, index=w965) -> (element=→"T3He2-2":dbl)
          }
          frame #6 {
            n549 = Search 1D Array(1D array=w973, element=T14."T3He3" ("SensorLocations")) -> (index of element=w970:i32)  [unwired: 1 in]
            n550 = Index Array(array=w971, index=w970) -> (element=→"T3He3":dbl)
          }
          frame #7 {
            n551 = Search 1D Array(1D array=w978, element=T14."T3He4" ("SensorLocations")) -> (index of element=w975:i32)  [unwired: 1 in]
            n552 = Index Array(array=w976, index=w975) -> (element=→"T3He4":dbl)
          }
          frame #8 {
            n553 = Search 1D Array(1D array=w983, element=T14."T3He5" ("SensorLocations")) -> (index of element=w980:i32)  [unwired: 1 in]
            n554 = Index Array(array=w981, index=w980) -> (element=→"T3He5":dbl)
          }
          frame #9 {
            n555 = Search 1D Array(1D array=w988, element=T14."T3He6-1" ("SensorLocations")) -> (index of element=w985:i32)  [unwired: 1 in]
            n556 = Index Array(array=w986, index=w985) -> (element=→"T3He6-1" →"T3He6-1/6-2 (HEX1)":dbl)
          }
          frame #10 {
            n557 = Search 1D Array(1D array=w993, element=T14."T3He6-2" ("SensorLocations")) -> (index of element=w990:i32)  [unwired: 1 in]
            n558 = Index Array(array=w991, index=w990) -> (element=→"T3He6-2" →"T3He6-1/6-2 (3He pot) 2":dbl)
          }
          frame #11 {
            n559 = Search 1D Array(1D array=w998, element=T14."T3He7-1" ("SensorLocations")) -> (index of element=w995:i32)  [unwired: 1 in]
            n560 = Index Array(array=w996, index=w995) -> (element=→"T3He7-1" →"T3He7-1/7-2 (HEX1)":dbl)
          }
          frame #12 {
            n561 = Search 1D Array(1D array=w1003, element=T14."T3He7-2" ("SensorLocations")) -> (index of element=w1000:i32)  [unwired: 1 in]
            n562 = Index Array(array=w1001, index=w1000) -> (element=→"T3He7-2" →"T3He7-1/6-2 (3He pot) 2":dbl)
          }
          frame #13 {
            n563 = Search 1D Array(1D array=w1008, element=T14."T3He8" ("SensorLocations")) -> (index of element=w1005:i32)  [unwired: 1 in]
            n564 = Index Array(array=w1006, index=w1005) -> (element=→"T3He8":dbl)
          }
          frame #14 {
            n565 = Search 1D Array(1D array=w1013, element=T14."T3He9" ("SensorLocations")) -> (index of element=w1010:i32)  [unwired: 1 in]
            n566 = Index Array(array=w1011, index=w1010) -> (element=→"T3He9":dbl)
          }
          frame #15 {
            n567 = Search 1D Array(1D array=w1018, element=T14."T3He10" ("SensorLocations")) -> (index of element=w1015:i32)  [unwired: 1 in]
            n568 = Index Array(array=w1016, index=w1015) -> (element=→"T3He10":dbl)
          }
          frame #16 {
            n569 = Search 1D Array(1D array=w1023, element=T14."T4He1" ("SensorLocations")) -> (index of element=w1020:i32)  [unwired: 1 in]
            n570 = Index Array(array=w1021, index=w1020) -> (element=→"T4He1" →"T4He1 (4K reservoir )":dbl)
          }
          frame #17 {
            n571 = Search 1D Array(1D array=w1028, element=T14."T4He2-1" ("SensorLocations")) -> (index of element=w1025:i32)  [unwired: 1 in]
            n572 = Index Array(array=w1026, index=w1025) -> (element=→"T4He2-1":dbl)
          }
          frame #18 {
            n573 = Search 1D Array(1D array=w1033, element=T14."T4He2-2" ("SensorLocations")) -> (index of element=w1030:i32)  [unwired: 1 in]
            n574 = Index Array(array=w1031, index=w1030) -> (element=→"T4He2-2":dbl)
          }
          frame #19 {
            n575 = Search 1D Array(1D array=w1038, element=T14."T4He3-1" ("SensorLocations")) -> (index of element=w1035:i32)  [unwired: 1 in]
            n576 = Index Array(array=w1036, index=w1035) -> (element=→"T4He3-1":dbl)
          }
          frame #20 {
            n577 = Search 1D Array(1D array=w1043, element=T14."T4He3-2" ("SensorLocations")) -> (index of element=w1040:i32)  [unwired: 1 in]
            n578 = Index Array(array=w1041, index=w1040) -> (element=→"T4He3-2":dbl)
          }
          frame #21 {
            n579 = Search 1D Array(1D array=w1048, element=T14."T4He3-3" ("SensorLocations")) -> (index of element=w1045:i32)  [unwired: 1 in]
            n580 = Index Array(array=w1046, index=w1045) -> (element=→"T4He3-3":dbl)
          }
          frame #22 {
            n581 = Search 1D Array(1D array=w1053, element=T14."T4He3-4" ("SensorLocations")) -> (index of element=w1050:i32)  [unwired: 1 in]
            n582 = Index Array(array=w1051, index=w1050) -> (element=→"T4He3-4":dbl)
          }
          frame #23 {
            n583 = Search 1D Array(1D array=w1058, element=T14."T4He4" ("SensorLocations")) -> (index of element=w1055:i32)  [unwired: 1 in]
            n584 = Index Array(array=w1056, index=w1055) -> (element=→"T4He4":dbl)
          }
          frame #24 {
            n585 = Search 1D Array(1D array=w1063, element=T14."T4He5" ("SensorLocations")) -> (index of element=w1060:i32)  [unwired: 1 in]
            n586 = Index Array(array=w1061, index=w1060) -> (element=→"T4He5":dbl)
          }
          frame #25 {
            n587 = Search 1D Array(1D array=w1068, element=T14."T4He6" ("SensorLocations")) -> (index of element=w1065:i32)  [unwired: 1 in]
            n588 = Index Array(array=w1066, index=w1065) -> (element=→"T4He6":dbl)
          }
          frame #26 {
            n589 = Search 1D Array(1D array=w1073, element=T14."T4He7" ("SensorLocations")) -> (index of element=w1070:i32)  [unwired: 1 in]
            n590 = Index Array(array=w1071, index=w1070) -> (element=→"T4He7":dbl)
          }
          frame #27 {
            n591 = Search 1D Array(1D array=w1078, element=T14."T4He8" ("SensorLocations")) -> (index of element=w1075:i32)  [unwired: 1 in]
            n592 = Index Array(array=w1076, index=w1075) -> (element=→"T4He8":dbl)
          }
          frame #28 {
            n593 = Search 1D Array(1D array=w1083, element=T14."T4He9" ("SensorLocations")) -> (index of element=w1080:i32)  [unwired: 1 in]
            n594 = Index Array(array=w1081, index=w1080) -> (element=→"T4He9":dbl)
          }
          frame #29 {
            n595 = Search 1D Array(1D array=w1088, element=T14."T4He10" ("SensorLocations")) -> (index of element=w1085:i32)  [unwired: 1 in]
            n596 = Index Array(array=w1086, index=w1085) -> (element=→"T4He10":dbl)
          }
          frame #30 {
            n597 = Search 1D Array(1D array=w1093, element=T14."T1K1" ("SensorLocations")) -> (index of element=w1090:i32)  [unwired: 1 in]
            n598 = Index Array(array=w1091, index=w1090) -> (element=→"T1K1":dbl)
          }
          frame #31 {
            n599 = Search 1D Array(1D array=w1098, element=T14."T1K2" ("SensorLocations")) -> (index of element=w1095:i32)  [unwired: 1 in]
            n600 = Index Array(array=w1096, index=w1095) -> (element=→"T1K2":dbl)
          }
          frame #32 {
            n601 = Search 1D Array(1D array=w1103, element=T14."T1K3-1" ("SensorLocations")) -> (index of element=w1100:i32)  [unwired: 1 in]
            n602 = Index Array(array=w1101, index=w1100) -> (element=→"T1K3-1" →"T1K3-1/3-2 (1K pot)":dbl)
          }
          frame #33 {
            n603 = Search 1D Array(1D array=w1108, element=T14."T1K3-2" ("SensorLocations")) -> (index of element=w1105:i32)  [unwired: 1 in]
            n604 = Index Array(array=w1106, index=w1105) -> (element=→"T1K3-2" →"T1K3-1/3-2 (1K pot) 2":dbl)
          }
          frame #34 {
            n605 = Search 1D Array(1D array=w1113, element=T14."T1K4" ("SensorLocations")) -> (index of element=w1110:i32)  [unwired: 1 in]
            n606 = Index Array(array=w1111, index=w1110) -> (element=→"T1K4":dbl)
          }
          frame #35 {
            n607 = Search 1D Array(1D array=w1118, element=T14."T1K5" ("SensorLocations")) -> (index of element=w1115:i32)  [unwired: 1 in]
            n608 = Index Array(array=w1116, index=w1115) -> (element=→"T1K5":dbl)
          }
          frame #36 {
            n609 = Search 1D Array(1D array=w1123, element=T14."T1K6" ("SensorLocations")) -> (index of element=w1120:i32)  [unwired: 1 in]
            n610 = Index Array(array=w1121, index=w1120) -> (element=→"T1K6":dbl)
          }
          frame #37 {
            n611 = Search 1D Array(1D array=w1128, element=T14."TIP1" ("SensorLocations")) -> (index of element=w1125:i32)  [unwired: 1 in]
            n612 = Index Array(array=w1126, index=w1125) -> (element=→"TIP1":dbl)
          }
          frame #38 {
            n613 = Search 1D Array(1D array=w1133, element=T14."TIP2" ("SensorLocations")) -> (index of element=w1130:i32)  [unwired: 1 in]
            n614 = Index Array(array=w1131, index=w1130) -> (element=→"TIP2":dbl)
          }
          frame #39 {
            n615 = Search 1D Array(1D array=w1138, element=T14."TIP3" ("SensorLocations")) -> (index of element=w1135:i32)  [unwired: 1 in]
            n616 = Index Array(array=w1136, index=w1135) -> (element=→"TIP3":dbl)
          }
          frame #40 {
            n617 = Search 1D Array(1D array=w1143, element=T14."TIP4" ("SensorLocations")) -> (index of element=w1140:i32)  [unwired: 1 in]
            n618 = Index Array(array=w1141, index=w1140) -> (element=→"TIP4":dbl)
          }
          frame #41 {
            n619 = Search 1D Array(1D array=w1148, element=T14."TIP5" ("SensorLocations")) -> (index of element=w1145:i32)  [unwired: 1 in]
            n620 = Index Array(array=w1146, index=w1145) -> (element=→"TIP5":dbl)
          }
          frame #42 {
            n621 = Search 1D Array(1D array=w1153, element=T14."TIP6" ("SensorLocations")) -> (index of element=w1150:i32)  [unwired: 1 in]
            n622 = Index Array(array=w1151, index=w1150) -> (element=→"TIP6":dbl)
          }
          frame #43 {
            n623 = Search 1D Array(1D array=w1158, element=T14."TIP7" ("SensorLocations")) -> (index of element=w1155:i32)  [unwired: 1 in]
            n624 = Index Array(array=w1156, index=w1155) -> (element=→"TIP7":dbl)
          }
          frame #44 {
            n625 = Search 1D Array(1D array=w1163, element=T14."TTH1" ("SensorLocations")) -> (index of element=w1160:i32)  [unwired: 1 in]
            n626 = Index Array(array=w1161, index=w1160) -> (element=→"TTH1":dbl)
          }
          frame #45 {
            n627 = Search 1D Array(1D array=w1168, element=T14."TTH2" ("SensorLocations")) -> (index of element=w1165:i32)  [unwired: 1 in]
            n628 = Index Array(array=w1166, index=w1165) -> (element=→"TTH2":dbl)
          }
          frame #46 {
            n629 = Search 1D Array(1D array=w1173, element=T14."TTH3" ("SensorLocations")) -> (index of element=w1170:i32)  [unwired: 1 in]
            n630 = Index Array(array=w1171, index=w1170) -> (element=→"TTH3":dbl)